vi "TLB Native Dynamic Events ver 0.26.vi"() -> ()   [LabVIEW 2018] (continued)
              shift-right: [w366] -> w361
              shift-left: w362 -> [w365]
              tunnel: string[] ["STOP", "RESET ENCODERS", "RESET YAW", "RESET ARM", "RESET ALL SENSORS", "DISPOSE CAM BUFFERS", "DISPOSE PROC BUFFERS", "CAM CLOSE", ""] -> [w364] mode=indexing
              n203 = Enqueue Element(queue=w365, element=w364) -> (queue out=w366:refnum<queue>)  [unwired: 2 in, 2 out]
            }
          }
          frame 4, Default {
            # ">>> Motor control cluster >>>"
            # ">>> yStepper command>>>"
            n204 = Dequeue Element(queue=w378, timeout in ms (-1)=w377, error in (no error)=w373) -> (element=w376:T8)  [unwired: 3 out]
            n205 = case shown="\"Start Task 5\"" w376 {
              tunnel: [w381 w389 w397 w405 w413 w421 w429 w437 w445 w452 w462 w470 w477 w480] -> w372
              tunnel: w375 -> [w382 w390 w398 w406 w414 w422 w430 w438 w446 w453 w461 w469 w477 w481]
              tunnel: [State_Type_Definitions,_for_0.26g_versions_and_later_2."Task 1A" ("Enum") State_Type_Definitions,_for_0.26g_versions_and_later_2."Task 2:Raise Arm" ("Enum") State_Type_Definitions,_for_0.26g_versions_and_later_2."Task 3" ("Enum") State_Type_Definitions,_for_0.26g_versions_and_later_2."Task 4_A" ("Enum") State_Type_Definitions,_for_0.26g_versions_and_later_2."Task 5A" ("Enum") State_Type_Definitions,_for_0.26g_versions_and_later_2."Task 6_A" ("Enum") State_Type_Definitions,_for_0.26g_versions_and_later_2."Task 8A: RAISE ARM" ("Enum") State_Type_Definitions,_for_0.26g_versions_and_later_2."Task 8A: RAISE ARM" ("Enum") State_Type_Definitions,_for_0.26g_versions_and_later_2."Task 8A: RAISE ARM" ("Enum") State_Type_Definitions,_for_0.26g_versions_and_later_2."Task 8A: RAISE ARM" ("Enum") State_Type_Definitions,_for_0.26g_versions_and_later_2."Task 9A: Raise Arm" ("Enum") State_Type_Definitions."Task 9F: SCAN IMAGE" ("Enum") State_Type_Definitions,_for_0.26g_versions_and_later_2."Idle" ("Enum") State_Type_Definitions,_for_0.26g_versions_and_later_2."Shutdown" ("Enum")] -> w374
              tunnel: [enum16{"Ball", "Soap", "Gel", "Pipe", "None"}."None" ("Object recognition mode") enum16{"Ball", "Soap", "Gel", "Pipe", "None"}."None" ("Object recognition mode") enum16{"Ball", "Soap", "Gel", "Pipe", "None"}."None" ("Object recognition mode") enum16{"Ball", "Soap", "Gel", "Pipe", "None"}."None" ("Object recognition mode") enum16{"Ball", "Soap", "Gel", "Pipe", "None"}."None" ("Object recognition mode") enum16{"Ball", "Soap", "Gel", "Pipe", "None"}."None" ("Object recognition mode") enum16{"Ball", "Soap", "Gel", "Pipe", "None"}."Ball" ("Object recognition mode") enum16{"Ball", "Soap", "Gel", "Pipe", "None"}."Gel" ("Object recognition mode") enum16{"Ball", "Soap", "Gel", "Pipe", "None"}."Pipe" ("Object recognition mode") enum16{"Ball", "Soap", "Gel", "Pipe", "None"}."Soap" ("Object recognition mode") enum16{"Ball", "Soap", "Gel", "Pipe", "None"}."None" ("Object recognition mode") enum16{"Ball", "Soap", "Gel", "Pipe", "None"}."None" ("Object recognition mode") enum16{"Ball", "Soap", "Gel", "Pipe", "None"}."None" ("Object recognition mode") enum16{"Ball", "Soap", "Gel", "Pipe", "None"}."None" ("Object recognition mode")] -> w367
              frame "Start Task 1" {
                n206 = for {
                  shift-right: [w386] -> w381
                  shift-left: w382 -> [w385]
                  tunnel: string[] ["RESET ENCODERS", "RESET YAW", "FORWARD", "READ ENCODERS"] -> [w384] mode=indexing
                  n207 = Enqueue Element(queue=w385, element=w384) -> (queue out=w386:refnum<queue>)  [unwired: 2 in, 2 out]
                }
              }
              frame "Start Task 2" {
                n208 = for {
                  shift-right: [w394] -> w389
                  shift-left: w390 -> [w393]
                  tunnel: string[] ["RESET ENCODERS", "RESET YAW", "READ ULTRASONIC", "ARDUINO - ULTRASONIC"] -> [w392] mode=indexing
                  n209 = Enqueue Element(queue=w393, element=w392) -> (queue out=w394:refnum<queue>)  [unwired: 2 in, 2 out]
                }
              }
              frame "Start Task 3" {
                n210 = for {
                  shift-right: [w402] -> w397
                  shift-left: w398 -> [w401]
                  tunnel: string[] ["RESET ENCODERS", "READ ENCODERS", "R-ACW"] -> [w400] mode=indexing
                  n211 = Enqueue Element(queue=w401, element=w400) -> (queue out=w402:refnum<queue>)  [unwired: 2 in, 2 out]
                }
              }
              frame "Start Task 4" {
                n212 = for {
                  shift-right: [w410] -> w405
                  shift-left: w406 -> [w409]
                  tunnel: string[] ["RESET YAW", "RESET ENCODERS", "RESET ARM", "RESET FLAGS", "", ""] -> [w408] mode=indexing
                  n213 = Enqueue Element(queue=w409, element=w408) -> (queue out=w410:refnum<queue>)  [unwired: 2 in, 2 out]
                }
              }
              frame "Start Task 5" {
                n214 = for {
                  shift-right: [w418] -> w413
                  shift-left: w414 -> [w417]
                  tunnel: string[] ["RESET YAW", "RESET ENCODERS", "RESET ARM", "RESET ALL SENSORS", "", ""] -> [w416] mode=indexing
                  n215 = Enqueue Element(queue=w417, element=w416) -> (queue out=w418:refnum<queue>)  [unwired: 2 in, 2 out]
                }
              }
              frame "Start Task 6" {
                n216 = for {
                  shift-right: [w426] -> w421
                  shift-left: w422 -> [w425]
                  tunnel: string[] ["OPEN LOG CAM ", "", "", "", "", ""] -> [w424] mode=indexing
                  n217 = Enqueue Element(queue=w425, element=w424) -> (queue out=w426:refnum<queue>)  [unwired: 2 in, 2 out]
                }
              }
              frame "Start Task 8 - BALL" {
                n218 = for {
                  shift-right: [w434] -> w429
                  shift-left: w430 -> [w433]
                  tunnel: string[] ["RESET YAW", "RESET ENCODERS", "RESET ARM", "RESET FLAGS"] -> [w432] mode=indexing
                  n219 = Enqueue Element(queue=w433, element=w432) -> (queue out=w434:refnum<queue>)  [unwired: 2 in, 2 out]
                }
              }
              frame "Start Task 8 - Gel" {
                n220 = for {
                  shift-right: [w442] -> w437
                  shift-left: w438 -> [w441]
                  tunnel: string[] ["RESET YAW", "RESET ENCODERS", "RESET ARM", "RESET FLAGS"] -> [w440] mode=indexing
                  n221 = Enqueue Element(queue=w441, element=w440) -> (queue out=w442:refnum<queue>)  [unwired: 2 in, 2 out]
                }
              }
              frame "Start Task 8 - Pipe" {
                n222 = for {
                  shift-right: [w450] -> w445
                  shift-left: w446 -> [w449]
                  tunnel: string[] ["RESET YAW", "RESET ENCODERS", "RESET ARM", "RESET FLAGS"] -> [w448] mode=indexing
                  n223 = Enqueue Element(queue=w449, element=w448) -> (queue out=w450:refnum<queue>)  [unwired: 2 in, 2 out]
                }
              }
              frame "Start Task 8 - Soap" {
                n224 = for {
                  shift-right: [w458] -> w452
                  shift-left: w453 -> [w457]
                  tunnel: string[] ["RESET YAW", "RESET ENCODERS", "RESET ARM", "RESET FLAGS"] -> [w456] mode=indexing
                  n225 = Enqueue Element(queue=w457, element=w456) -> (queue out=w458:refnum<queue>)  [unwired: 2 in, 2 out]
                }
              }
              frame "Start Task 9" {
                n226 = for {
                  shift-right: [w466] -> w462
                  shift-left: w461 -> [w465]
                  tunnel: string[] ["RESET ENCODERS", "READ ENCODERS", "Z STEPPER BOX HEIGHT"] -> [w464] mode=indexing
                  n227 = Enqueue Element(queue=w465, element=w464) -> (queue out=w466:refnum<queue>)  [unwired: 2 in, 2 out]
                }
              }
              frame "Start Task A" {
                n228 = for {
                  shift-right: [w474] -> w470
                  shift-left: w469 -> [w473]
                  tunnel: string[] ["RESET ENCODERS", "READ ENCODERS", "RESET YAW", "Z STEPPER BOX HEIGHT"] -> [w472] mode=indexing
                  n229 = Enqueue Element(queue=w473, element=w472) -> (queue out=w474:refnum<queue>)  [unwired: 2 in, 2 out]
                }
              }
              frame "None", Default {
              }
              frame "Exit" {
                n230 = for {
                  shift-right: [w485] -> w480
                  shift-left: w481 -> [w484]
                  tunnel: string[] ["STOP", "RESET ENCODERS", "RESET YAW", "EXIT"] -> [w483] mode=indexing
                  n231 = Enqueue Element(queue=w484, element=w483) -> (queue out=w485:refnum<queue>)  [unwired: 2 in, 2 out]
                }
              }
            }
          }
          frame 5 {
            # ">> Item Selection Bias >>"
            # ">>> yStepper command>>>"
            n232 = for {
              shift-right: [w496] -> w490
              shift-left: w492 -> [w495]
              tunnel: string[] ["INIT", "RESET ENCODERS", "RESET FLAGS", "CAM CLOSE", "DISPOSE BUFFERS", "EXIT", ""] -> [w494] mode=indexing
              n233 = Enqueue Element(queue=w495, element=w494) -> (queue out=w496:refnum<queue>)  [unwired: 2 in, 2 out]
            }
          }
          frame 6 {
            # ">>> Motor control cluster >>>"
            # ">> Line detection >>"
            # ">> Checks if 1 metre moved >>"
            # ">>> yStepper command>>>"
            # "Use 250"
            n234 = Greater?(x=w506, y=265.0) -> (0:w500:bool)
            n235 = Dequeue Element(queue=w513, timeout in ms (-1)=w512, error in (no error)=w511) -> (element=w510:T8)  [unwired: 3 out]
            n236 = And(x=w499, y=w500) -> (x .and. y?=w497:bool)
            n237 = case shown="\"Start Task 1\", Default" w510 {
              tunnel: w498 -> [w514 _]
              tunnel: [w524 State_Type_Definitions,_for_0.26g_versions_and_later_2."True Stop" ("Enum")] -> w509
              tunnel: w508 -> [w522 w539]
              tunnel: [w521 w538] -> w507
              tunnel: [State_Type_Definitions,_for_0.26g_versions_and_later_2."Idle" ("Enum") State_Type_Definitions,_for_0.26g_versions_and_later_2."Shutdown" ("Enum")] -> w504
              tunnel: w497 -> [w515 _]
              frame "Start Task 1", Default {
                n238 = Or(x=w515, y=w514) -> (x .or. y?=w516:bool)
                n239 = case shown="True" w516 {
                  tunnel: w522 -> [w527 w533]
                  tunnel: [w526 w531] -> w521
                  frame False {
                    n240 = for {
                      shift-right: [w529] -> w526
                      shift-left: w527 -> [w530]
                      tunnel: string[] ["READ ENCODERS", "READ NAVX", "FORWARD", "READ LINE SENSOR"] ("element") -> [w528] mode=indexing
                      n241 = Enqueue Element(queue=w530, element=w528) -> (queue out=w529:refnum<queue>)  [unwired: 2 in, 2 out]
                    }
                  }
                  frame True {
                    n242 = for {
                      shift-right: [w535] -> w531
                      shift-left: w533 -> [w536]
                      tunnel: string[] ["RESET YAW", "RESET ENCODERS", "STOP", ""] -> [w534] mode=indexing
                      n243 = Enqueue Element(queue=w536, element=w534) -> (queue out=w535:refnum<queue>)  [unwired: 2 in, 2 out]
                    }
                  }
                }
                n244 = Select(t=State_Type_Definitions,_for_0.26g_versions_and_later_2."True Stop" ("Enum"), s=w514, f=State_Type_Definitions,_for_0.26g_versions_and_later_2."Task 1B" ("Enum")) -> (s? t:f=w519:T16)
                n245 = Select(t=w519, s=w515, f=State_Type_Definitions,_for_0.26g_versions_and_later_2."Task 1A" ("Enum")) -> (s? t:f=w524:T16)
              }
              frame "Exit" {
                n246 = for {
                  shift-right: [w543] -> w538
                  shift-left: w539 -> [w544]
                  tunnel: string[] ["STOP", "RESET ENCODERS", "RESET YAW", ""] -> [w542] mode=indexing
                  n247 = Enqueue Element(queue=w544, element=w542) -> (queue out=w543:refnum<queue>)  [unwired: 2 in, 2 out]
                }
              }
            }
          }
          frame 7 {
            # ">>> Motor control cluster >>>"
            # ">> Line detection >>"
            # ">> Adds small distance overhead after 1M >>"
            # ">>> yStepper command>>>"
            n248 = Greater?(x=w551, y=50.0) -> (0:w545:bool)
            n249 = Dequeue Element(queue=w560, timeout in ms (-1)=w559, error in (no error)=w558) -> (element=w557:T8)  [unwired: 3 out]
            n250 = Or(x=w545, y=w552) -> (x .or. y?=w556:bool)
            n251 = case shown="\"Start Task 1\", Default" w557 {
              tunnel: w556 -> [w563 _]
              tunnel: [w567 State_Type_Definitions,_for_0.26g_versions_and_later_2."True Stop" ("Enum")] -> w555
              tunnel: w554 -> [w564 w582]
              tunnel: [w562 w581] -> w553
              tunnel: [State_Type_Definitions,_for_0.26g_versions_and_later_2."Idle" ("Enum") State_Type_Definitions,_for_0.26g_versions_and_later_2."Shutdown" ("Enum")] -> w549
              frame "Start Task 1", Default {
                n252 = case shown="True" w563 {
                  tunnel: w564 -> [w570 w576]
                  tunnel: [w569 w574] -> w562
                  frame False {
                    n253 = for {
                      shift-right: [w572] -> w569
                      shift-left: w570 -> [w573]
                      tunnel: string[] ["READ ENCODERS", "READ NAVX", "FORWARD", "READ LINE SENSOR"] ("element") -> [w571] mode=indexing
                      n254 = Enqueue Element(queue=w573, element=w571) -> (queue out=w572:refnum<queue>)  [unwired: 2 in, 2 out]
                    }
                  }
                  frame True {
                    n255 = for {
                      shift-right: [w578] -> w574
                      shift-left: w576 -> [w579]
                      tunnel: string[] ["RESET YAW", "RESET ENCODERS", "STOP", ""] -> [w577] mode=indexing
                      n256 = Enqueue Element(queue=w579, element=w577) -> (queue out=w578:refnum<queue>)  [unwired: 2 in, 2 out]
                    }
                  }
                }
                n257 = Select(t=State_Type_Definitions,_for_0.26g_versions_and_later_2."True Stop" ("Enum"), s=w563, f=State_Type_Definitions,_for_0.26g_versions_and_later_2."Task 1B" ("Enum")) -> (s? t:f=w567:T16)
              }
              frame "Exit" {
                n258 = for {
                  shift-right: [w586] -> w581
                  shift-left: w582 -> [w587]
                  tunnel: string[] ["STOP", "RESET ENCODERS", "RESET YAW", ""] -> [w585] mode=indexing
                  n259 = Enqueue Element(queue=w587, element=w585) -> (queue out=w586:refnum<queue>)  [unwired: 2 in, 2 out]
                }
              }
            }
          }
          frame 8 {
            # ">> Stepper height reeached >>"
            # ">>> yStepper command>>>"
            # ">> Manual override >>"
            n260 = Dequeue Element(queue=w593, timeout in ms (-1)=w592, error in (no error)=w591) -> (element=w602:T8)  [unwired: 3 out]
            n261 = Equal?(x=w595, y=u8 60) -> (x = y?=w600:bool)
            n262 = case shown="\"Start Task 1\", Default" w602 {
              tunnel: [w613 State_Type_Definitions,_for_0.26g_versions_and_later_2."True Stop" ("Enum")] -> w597
              tunnel: [w611 w628] -> w590
              tunnel: w599 -> [w610 _]
              tunnel: w598 -> [w604 _]
              tunnel: [State_Type_Definitions,_for_0.26g_versions_and_later_2."Idle" ("Enum") State_Type_Definitions,_for_0.26g_versions_and_later_2."Shutdown" ("Enum")] -> w596
              tunnel: w600 -> [w603 _]
              frame "Start Task 1", Default {
                # ">> WIill proceed to part ii if not manual override >>"
                # ">>If ENABLE or Trigger is set to true>>"
                n263 = Or(x=w603, y=w604) -> (x .or. y?=w605:bool)
                n264 = case shown="True" w603 {
                  tunnel: [w616 w622] -> w611
                  tunnel: w610 -> [w615 w621]
                  frame False {
                    n265 = for {
                      shift-right: [w618] -> w616
                      shift-left: w615 -> [w619]
                      tunnel: string[] ["Z STEPPER CAM HEIGHT", "READ STEPPER VALUES"] ("element") -> [w617] mode=indexing
                      n266 = Enqueue Element(queue=w619, element=w617) -> (queue out=w618:refnum<queue>)  [unwired: 2 in, 2 out]
                    }
                  }
                  frame True {
                    n267 = for {
                      shift-right: [w624] -> w622
                      shift-left: w621 -> [w625]
                      tunnel: string[] ["ARDUINO - ULTRASONIC", "READ ULTRASONIC", "", "", "", ""] -> [w623] mode=indexing
                      n268 = Enqueue Element(queue=w625, element=w623) -> (queue out=w624:refnum<queue>)  [unwired: 2 in, 2 out]
                    }
                  }
                }
                n269 = Select(t=State_Type_Definitions,_for_0.26g_versions_and_later_2."True Stop" ("Enum"), s=w604, f=State_Type_Definitions,_for_0.26g_versions_and_later_2."Task 2:Sensor Mode" ("Enum")) -> (s? t:f=w607:T16)
                n270 = Select(t=w607, s=w605, f=State_Type_Definitions,_for_0.26g_versions_and_later_2."Task 2:Raise Arm" ("Enum")) -> (s? t:f=w613:T16)
              }
              frame "Exit" {
                n271 = for {
                  shift-right: [w631] -> w628
                  shift-left: _ -> [w632]
                  tunnel: string[] ["STOP", "RESET ENCODERS", "RESET YAW", ""] -> [w630] mode=indexing
                  n272 = Enqueue Element(queue=w632, element=w630) -> (queue out=w631:refnum<queue>)  [unwired: 2 in, 2 out]
                }
              }
            }
          }
          frame 9 {
            w649 = u8 20 ("y")
            # ">>> yStepper command>>>"
            # ">>Object detected>>"
            n273 = Dequeue Element(queue=w642, timeout in ms (-1)=w641, error in (no error)=w640) -> (element=w650:T8)  [unwired: 3 out]
            n274 = Less?(x=w638, y=w649) -> (x < y?=w648:bool)
            n275 = Less?(x=w637, y=w649) -> (x < y?=w647:bool)
            n276 = Or(x=w648, y=w647) -> (x .or. y?=w633:bool)
            n277 = case shown="\"Start Task 1\", Default" w650 {
              tunnel: w633 -> [w653 _]
              tunnel: [w660 State_Type_Definitions,_for_0.26g_versions_and_later_2."True Stop" ("Enum")] -> w646
              tunnel: w639 -> [w652 _]
              tunnel: w643 -> [w659 w676]
              tunnel: [w658 w677] -> w645
              tunnel: [State_Type_Definitions,_for_0.26g_versions_and_later_2."Idle" ("Enum") State_Type_Definitions,_for_0.26g_versions_and_later_2."Shutdown" ("Enum")] -> w644
              frame "Start Task 1", Default {
                n278 = case shown="False" w653 {
                  tunnel: w659 -> [w663 w670]
                  tunnel: [w664 w669] -> w658
                  frame False {
                    n279 = for {
                      tunnel: string[] ["READ ULTRASONIC", "STOP"] ("element") -> [w665] mode=indexing
                      shift-right: [w667] -> w664
                      shift-left: w663 -> [w666]
                      n280 = Enqueue Element(queue=w666, element=w665) -> (queue out=w667:refnum<queue>)  [unwired: 2 in, 2 out]
                    }
                  }
                  frame True {
                    n281 = for {
                      shift-right: [w672] -> w669
                      shift-left: w670 -> [w673]
                      tunnel: string[] ["RESET ENCODERS", "READ NAVX", "READ ENCODERS"] -> [w671] mode=indexing
                      n282 = Enqueue Element(queue=w673, element=w671) -> (queue out=w672:refnum<queue>)  [unwired: 2 in, 2 out]
                    }
                  }
                }
                n283 = Or(x=w653, y=w652) -> (x .or. y?=w651:bool)
                n284 = Select(t=State_Type_Definitions,_for_0.26g_versions_and_later_2."True Stop" ("Enum"), s=w652, f=State_Type_Definitions,_for_0.26g_versions_and_later_2."Task 2:Reverse Mode" ("Enum")) -> (s? t:f=w654:T16)
                n285 = Select(t=w654, s=w651, f=State_Type_Definitions,_for_0.26g_versions_and_later_2."Task 2:Sensor Mode" ("Enum")) -> (s? t:f=w660:T16)
              }
              frame "Exit" {
                n286 = for {
                  shift-right: [w680] -> w677
                  shift-left: w676 -> [w681]
                  tunnel: string[] ["STOP", "RESET ENCODERS", "RESET YAW", "ARDUINO MODE 0"] -> [w679] mode=indexing
                  n287 = Enqueue Element(queue=w681, element=w679) -> (queue out=w680:refnum<queue>)  [unwired: 2 in, 2 out]
                }
              }
            }
          }
          frame 10 {
            # ">>> yStepper command>>>"
            n288 = Dequeue Element(queue=w692, timeout in ms (-1)=w693, error in (no error)=w694) -> (element=w696:T8)  [unwired: 3 out]
            n289 = Less?(x=w686, y=-50.0) -> (x < y?=w684:bool)
            n290 = case shown="\"Start Task 1\", Default" w696 {
              tunnel: [w706 State_Type_Definitions,_for_0.26g_versions_and_later_2."True Stop" ("Enum")] -> w688
              tunnel: w695 -> [w699 _]
              tunnel: w691 -> [w705 w722]
              tunnel: [w704 w723] -> w687
              tunnel: [State_Type_Definitions,_for_0.26g_versions_and_later_2."Idle" ("Enum") State_Type_Definitions,_for_0.26g_versions_and_later_2."Shutdown" ("Enum")] -> w689
              tunnel: w684 -> [w697 _]
              frame "Start Task 1", Default {
                n291 = case shown="True" w697 {
                  tunnel: w705 -> [w709 w716]
                  tunnel: [w710 w715] -> w704
                  frame False {
                    n292 = for {
                      tunnel: string[] ["READ ENCODERS", "REVERSE", "READ NAVX"] ("element") -> [w711] mode=indexing
                      shift-right: [w713] -> w710
                      shift-left: w709 -> [w712]
                      n293 = Enqueue Element(queue=w712, element=w711) -> (queue out=w713:refnum<queue>)  [unwired: 2 in, 2 out]
                    }
                  }
                  frame True {
                    n294 = for {
                      shift-right: [w718] -> w715
                      shift-left: w716 -> [w719]
                      tunnel: string[] ["STOP", "ARDUINO - ULTRASONIC", "READ ULTRASONIC", "RESET ENCODERS"] -> [w717] mode=indexing
                      n295 = Enqueue Element(queue=w719, element=w717) -> (queue out=w718:refnum<queue>)  [unwired: 2 in, 2 out]
                    }
                  }
                }
                n296 = Or(x=w697, y=w699) -> (x .or. y?=w698:bool)
                n297 = Select(t=State_Type_Definitions,_for_0.26g_versions_and_later_2."True Stop" ("Enum"), s=w699, f=State_Type_Definitions,_for_0.26g_versions_and_later_2."Task 2:Sensor Mode" ("Enum")) -> (s? t:f=w700:T16)
                n298 = Select(t=w700, s=w698, f=State_Type_Definitions,_for_0.26g_versions_and_later_2."Task 2:Reverse Mode" ("Enum")) -> (s? t:f=w706:T16)
              }
              frame "Exit" {
                n299 = for {
                  shift-right: [w726] -> w723
                  shift-left: w722 -> [w727]
                  tunnel: string[] ["STOP", "RESET ENCODERS", "RESET YAW", "ARDUINO MODE 0"] -> [w725] mode=indexing
                  n300 = Enqueue Element(queue=w727, element=w725) -> (queue out=w726:refnum<queue>)  [unwired: 2 in, 2 out]
                }
              }
            }
          }
          frame 11 {
            # ">>> Motor control cluster >>>"
            # ">>> yStepper command>>>"
            n301 = Dequeue Element(queue=w743, timeout in ms (-1)=w742, error in (no error)=w741) -> (element=w732:T8)  [unwired: 3 out]
            n302 = Less?(x=w740, y=-160.0) -> (x < y?=w737:bool)
            n303 = Or(x=w737, y=w738) -> (x .or. y?=w733:bool)
            n304 = case shown="\"Start Task 1\", Default" w732 {
              tunnel: w733 -> [w746 _]
              tunnel: [w750 State_Type_Definitions,_for_0.26g_versions_and_later_2."True Stop" ("Enum")] -> w734
              tunnel: w736 -> [w747 w766]
              tunnel: [w745 w765] -> w735
              tunnel: [State_Type_Definitions,_for_0.26g_versions_and_later_2."Idle" ("Enum") State_Type_Definitions,_for_0.26g_versions_and_later_2."Shutdown" ("Enum")] -> w731
              frame "Start Task 1", Default {
                n305 = case shown="False" w746 {
                  tunnel: w747 -> [w753 w759]
                  tunnel: [w752 w757] -> w745
                  frame False {
                    n306 = for {
                      shift-right: [w755] -> w752
                      shift-left: w753 -> [w756]
                      tunnel: string[] ["READ ENCODERS", "R-CW"] ("element") -> [w754] mode=indexing
                      n307 = Enqueue Element(queue=w756, element=w754) -> (queue out=w755:refnum<queue>)  [unwired: 2 in, 2 out]
                    }
                  }
                  frame True {
                    n308 = for {
                      shift-right: [w761] -> w757
                      shift-left: w759 -> [w762]
                      tunnel: string[] ["RESET YAW", "RESET ENCODERS", "STOP", "ARDUINO MODE 0"] -> [w760] mode=indexing
                      n309 = Enqueue Element(queue=w762, element=w760) -> (queue out=w761:refnum<queue>)  [unwired: 2 in, 2 out]
                    }
                  }
                }
                n310 = Select(t=State_Type_Definitions,_for_0.26g_versions_and_later_2."True Stop" ("Enum"), s=w746, f=State_Type_Definitions,_for_0.26g_versions_and_later_2."Task 3" ("Enum")) -> (s? t:f=w750:T16)
              }
              frame "Exit" {
                n311 = for {
                  shift-right: [w769] -> w765
                  shift-left: w766 -> [w770]
                  tunnel: string[] ["STOP", "RESET ENCODERS", "RESET YAW", ""] -> [w768] mode=indexing
                  n312 = Enqueue Element(queue=w770, element=w768) -> (queue out=w769:refnum<queue>)  [unwired: 2 in, 2 out]
                }
              }
            }
          }
          frame 12 {
            # ">> Stepper height reeached >>"
            # ">>> yStepper command>>>"
            # ">> Manual override >>"
            n313 = Dequeue Element(queue=w784, timeout in ms (-1)=w783, error in (no error)=w782) -> (element=w781:T8)  [unwired: 3 out]
            n314 = Equal?(x=w775, y=u8 60) -> (x = y?=w773:bool)
            n315 = case shown="\"Start Task 1\", Default" w781 {
              tunnel: [w796 State_Type_Definitions,_for_0.26g_versions_and_later_2."True Stop" ("Enum")] -> w780
              tunnel: [w794 w812] -> w779
              tunnel: w785 -> [w793 w809]
              tunnel: w778 -> [w787 _]
              tunnel: [State_Type_Definitions,_for_0.26g_versions_and_later_2."Idle" ("Enum") State_Type_Definitions,_for_0.26g_versions_and_later_2."Shutdown" ("Enum")] -> w777
              tunnel: w773 -> [w786 _]
              frame "Start Task 1", Default {
                # ">> WIill proceed to part ii if not manual override >>"
                # ">>If ENABLE or Trigger is set to true>>"
                n316 = Or(x=w786, y=w787) -> (x .or. y?=w788:bool)
                n317 = case shown="False" w786 {
                  tunnel: [w799 w805] -> w794
                  tunnel: w793 -> [w798 w804]
                  frame False {
                    n318 = for {
                      shift-right: [w801] -> w799
                      shift-left: w798 -> [w802]
                      tunnel: string[] ["Z STEPPER CAM HEIGHT", "READ STEPPER VALUES"] ("element") -> [w800] mode=indexing
                      n319 = Enqueue Element(queue=w802, element=w800) -> (queue out=w801:refnum<queue>)  [unwired: 2 in, 2 out]
                    }
                  }
                  frame True {
                    n320 = for {
                      shift-right: [w807] -> w805
                      shift-left: w804 -> [w808]
                      tunnel: string[] ["ARDUINO - ULTRASONIC", "READ ULTRASONIC", "FORWARD", "", "", ""] -> [w806] mode=indexing
                      n321 = Enqueue Element(queue=w808, element=w806) -> (queue out=w807:refnum<queue>)  [unwired: 2 in, 2 out]
                    }
                  }
                }
                n322 = Select(t=State_Type_Definitions,_for_0.26g_versions_and_later_2."True Stop" ("Enum"), s=w787, f=State_Type_Definitions,_for_0.26g_versions_and_later_2."Task 4_B" ("Enum")) -> (s? t:f=w790:T16)
                n323 = Select(t=w790, s=w788, f=State_Type_Definitions,_for_0.26g_versions_and_later_2."Task 4_A" ("Enum")) -> (s? t:f=w796:T16)
              }
              frame "Exit" {
                n324 = for {
                  shift-right: [w815] -> w812
                  shift-left: w809 -> [w816]
                  tunnel: string[] ["STOP", "RESET ENCODERS", "RESET YAW", ""] -> [w814] mode=indexing
                  n325 = Enqueue Element(queue=w816, element=w814) -> (queue out=w815:refnum<queue>)  [unwired: 2 in, 2 out]
                }
              }
            }
          }
          frame 13 {
            w822 = u8 20
            # ">> Path blocked >>"
            # ">>> yStepper command>>>"
            # ">> Manual override >>"
            n326 = Dequeue Element(queue=w831, timeout in ms (-1)=w830, error in (no error)=w829) -> (element=w828:T8)  [unwired: 3 out]
            n327 = Less?(x=w824, y=w822) -> (x < y?=w819:bool)
            n328 = Less?(x=w823, y=w822) -> (x < y?=w820:bool)
            n329 = And(x=w820, y=w819) -> (x .and. y?=w821:bool)
            n330 = case shown="\"Start Task 1\", Default" w828 {
              tunnel: [w845 State_Type_Definitions,_for_0.26g_versions_and_later_2."True Stop" ("Enum")] -> w833
              tunnel: [w843 w860] -> w834
              tunnel: w827 -> [w842 _]
              tunnel: w832 -> [w836 _]
              tunnel: [State_Type_Definitions,_for_0.26g_versions_and_later_2."Idle" ("Enum") State_Type_Definitions,_for_0.26g_versions_and_later_2."Shutdown" ("Enum")] -> w826
              tunnel: w821 -> [w835 _]
              frame "Start Task 1", Default {
                # ">> Manual override forces program to true stop >>"
                # ">>If ENABLE or Trigger is set to true>>"
                n331 = Or(x=w835, y=w836) -> (x .or. y?=w841:bool)
                n332 = case shown="False" w835 {
                  tunnel: [w848 w853] -> w843
                  tunnel: w842 -> [w847 w852]
                  frame False {
                    n333 = for {
                      shift-right: [w850] -> w848
                      shift-left: w847 -> [w851]
                      tunnel: string[] ["FORWARD", "READ ULTRASONIC", "READ NAVX"] ("element") -> [w849] mode=indexing
                      n334 = Enqueue Element(queue=w851, element=w849) -> (queue out=w850:refnum<queue>)  [unwired: 2 in, 2 out]
                    }
                  }
                  frame True {
                    n335 = for {
                      shift-right: [w856] -> w853
                      shift-left: w852 -> [w857]
                      tunnel: string[] ["STOP", "RESET YAW", "RESET ENCODERS", "RESET FLAGS"] -> [w855] mode=indexing
                      n336 = Enqueue Element(queue=w857, element=w855) -> (queue out=w856:refnum<queue>)  [unwired: 2 in, 2 out]
                    }
                  }
                }
                n337 = Select(t=State_Type_Definitions,_for_0.26g_versions_and_later_2."True Stop" ("Enum"), s=w836, f=State_Type_Definitions,_for_0.26g_versions_and_later_2."Task 4_C" ("Enum")) -> (s? t:f=w838:T16)
                n338 = Select(t=w838, s=w841, f=State_Type_Definitions,_for_0.26g_versions_and_later_2."Task 4_B" ("Enum")) -> (s? t:f=w845:T16)
              }
              frame "Exit" {
                n339 = for {
                  shift-right: [w863] -> w860
                  shift-left: _ -> [w864]
                  tunnel: string[] ["STOP", "RESET ENCODERS", "RESET YAW", ""] -> [w862] mode=indexing
                  n340 = Enqueue Element(queue=w864, element=w862) -> (queue out=w863:refnum<queue>)  [unwired: 2 in, 2 out]
                }
              }
            }
          }
          frame 14 {
            w876 = u8 20
            # ">> xDistance travelled>>"
            # ">> Path NOT blocked >>"
            # ">>> yStepper command>>>"
            # ">> Manual override >>"
            n341 = Dequeue Element(queue=w886, timeout in ms (-1)=w879, error in (no error)=w878) -> (element=w880:T8)  [unwired: 3 out]
            n342 = Greater?(x=w868, y=w876) -> (0:w874:bool)
            n343 = Greater?(x=w873, y=80.0) -> (0:w871:bool)
            n344 = Greater?(x=w867, y=w876) -> (0:w875:bool)
            n345 = And(x=w875, y=w874) -> (x .and. y?=w870:bool)
            n346 = And(x=w871, y=w870) -> (x .and. y?=w869:bool)
            n347 = case shown="\"Start Task 1\", Default" w880 {
              tunnel: [w897 State_Type_Definitions,_for_0.26g_versions_and_later_2."True Stop" ("Enum")] -> w883
              tunnel: [w895 w913] -> w882
              tunnel: w885 -> [w894 w910]
              tunnel: w884 -> [w888 _]
              tunnel: [State_Type_Definitions,_for_0.26g_versions_and_later_2."Idle" ("t") State_Type_Definitions,_for_0.26g_versions_and_later_2."Shutdown" ("Enum")] -> w881
              tunnel: w869 -> [w887 _]
              frame "Start Task 1", Default {
                # ">> Manual override forces program to true stop >>"
                # ">>If ENABLE or Trigger is set to true>>"
                n348 = Or(x=w887, y=w888) -> (x .or. y?=w893:bool)
                n349 = case shown="False" w887 {
                  tunnel: [w900 w905] -> w895
                  tunnel: w894 -> [w898 w904]
                  frame False {
                    n350 = for {
                      shift-right: [w902] -> w900
                      shift-left: w898 -> [w903]
                      tunnel: string[] ["RIGHT", "READ NAVX", "READ ENCODERS", "READ ULTRASONIC"] ("element") -> [w901] mode=indexing
                      n351 = Enqueue Element(queue=w903, element=w901) -> (queue out=w902:refnum<queue>)  [unwired: 2 in, 2 out]
                    }
                  }
                  frame True {
                    n352 = for {
                      shift-right: [w908] -> w905
                      shift-left: w904 -> [w909]
                      tunnel: string[] ["STOP", "RESET YAW", "RESET ENCODERS", "ARDUINO - ULTRASONIC"] -> [w907] mode=indexing
                      n353 = Enqueue Element(queue=w909, element=w907) -> (queue out=w908:refnum<queue>)  [unwired: 2 in, 2 out]
                    }
                  }
                }
                n354 = Select(t=State_Type_Definitions,_for_0.26g_versions_and_later_2."True Stop" ("Enum"), s=w888, f=State_Type_Definitions,_for_0.26g_versions_and_later_2."Task 4_D" ("Enum")) -> (s? t:f=w889:T16)
                n355 = Select(t=w889, s=w893, f=State_Type_Definitions,_for_0.26g_versions_and_later_2."Task 4_C" ("Enum")) -> (s? t:f=w897:T16)
              }
              frame "Exit" {
                n356 = for {
                  shift-right: [w916] -> w913
                  shift-left: w910 -> [w917]
                  tunnel: string[] ["STOP", "RESET ENCODERS", "RESET YAW", ""] -> [w915] mode=indexing
                  n357 = Enqueue Element(queue=w917, element=w915) -> (queue out=w916:refnum<queue>)  [unwired: 2 in, 2 out]
                }
              }
            }
          }
          frame 15 {
            w940 = u8 20
            # ">>> Motor control cluster >>>"
            # ">> Line detected >>"
            # ">> yDistance travelled>>"
            # ">> Path blocked >>"
            # ">>> yStepper command>>>"
            # ">> Manual override >>"
            n358 = Less?(x=w925, y=w940) -> (x < y?=w938:bool)
            n359 = Greater?(x=w929, y=200.0) -> (0:w936:bool)
            n360 = Less?(x=w924, y=w940) -> (x < y?=w939:bool)
            n361 = And(x=w939, y=w938) -> (x .and. y?=w935:bool)
            n362 = Dequeue Element(queue=w932, timeout in ms (-1)=w931, error in (no error)=w930) -> (element=w941:T8)  [unwired: 3 out]
            n363 = Or(x=w936, y=w935) -> (x .or. y?=w919:bool)
            n364 = And(x=w920, y=w919) -> (x .and. y?=w918:bool)
            n365 = case shown="\"Start Task 1\", Default" w941 {
              tunnel: [w952 State_Type_Definitions,_for_0.26g_versions_and_later_2."True Stop" ("Enum")] -> w928
              tunnel: [w950 w968] -> w926
              tunnel: w933 -> [w949 w965]
              tunnel: w934 -> [w943 _]
              tunnel: [State_Type_Definitions,_for_0.26g_versions_and_later_2."Idle" ("t") State_Type_Definitions,_for_0.26g_versions_and_later_2."Shutdown" ("Enum")] -> w927
              tunnel: w918 -> [w942 _]
              frame "Start Task 1", Default {
                # ">> Manual override forces program to true stop >>"
                # ">>If ENABLE or Trigger is set to true>>"
                n366 = Or(x=w942, y=w943) -> (x .or. y?=w948:bool)
                n367 = case shown="False" w942 {
                  tunnel: [w955 w960] -> w950
                  tunnel: w949 -> [w953 w959]
                  frame False {
                    n368 = for {
                      shift-right: [w957] -> w955
                      shift-left: w953 -> [w958]
                      tunnel: string[] ["FORWARD", "READ NAVX", "READ ENCODERS", "READ ULTRASONIC", "READ LINE SENSOR"] ("element") -> [w956] mode=indexing
                      n369 = Enqueue Element(queue=w958, element=w956) -> (queue out=w957:refnum<queue>)  [unwired: 2 in, 2 out]
                    }
                  }
                  frame True {
                    n370 = for {
                      shift-right: [w963] -> w960
                      shift-left: w959 -> [w964]
                      tunnel: string[] ["STOP", "RESET YAW", "RESET ENCODERS", "RESET FLAGS"] -> [w962] mode=indexing
                      n371 = Enqueue Element(queue=w964, element=w962) -> (queue out=w963:refnum<queue>)  [unwired: 2 in, 2 out]
                    }
                  }
                }
                n372 = Select(t=State_Type_Definitions,_for_0.26g_versions_and_later_2."True Stop" ("Enum"), s=w943, f=State_Type_Definitions,_for_0.26g_versions_and_later_2."True Stop" ("Enum")) -> (s? t:f=w944:T16)
                n373 = Select(t=w944, s=w948, f=State_Type_Definitions,_for_0.26g_versions_and_later_2."Task 4_D" ("Enum")) -> (s? t:f=w952:T16)
              }
              frame "Exit" {
                n374 = for {
                  shift-right: [w971] -> w968
                  shift-left: w965 -> [w972]
                  tunnel: string[] ["STOP", "RESET ENCODERS", "RESET YAW", ""] -> [w970] mode=indexing
                  n375 = Enqueue Element(queue=w972, element=w970) -> (queue out=w971:refnum<queue>)  [unwired: 2 in, 2 out]
                }
              }
            }
          }
          frame 16 {
            # "Stays in Task 5_A until stepper reaches desired \nheight"
            # ">>> Motor control cluster >>>"
            # ">>> yStepper command>>>"
            # ">> Manual override >>"
            n376 = Dequeue Element(queue=w983, timeout in ms (-1)=w982, error in (no error)=w984) -> (element=w981:T8)  [unwired: 3 out]
            n377 = Equal?(x=w980, y=u8 1) -> (x = y?=w978:bool)
            n378 = case shown="\"Start Task 1\", Default" w981 {
              tunnel: [w994 State_Type_Definitions,_for_0.26g_versions_and_later_2."True Stop" ("Enum")] -> w985
              tunnel: [w997 w1014] -> w986
              tunnel: [State_Type_Definitions,_for_0.26g_versions_and_later_2."Idle" ("Enum") State_Type_Definitions,_for_0.26g_versions_and_later_2."Shutdown" ("Enum")] -> w987
              tunnel: w978 -> [w993 _]
              tunnel: w977 -> [w992 _]
              tunnel: w976 -> [w988 w1011]
              frame "Start Task 1", Default {
                # "T: Go back to idle, F: Continue with task\""
                # ">> Manual override >>"
                n379 = case shown="True" w993 {
                  tunnel: [w1001 w1007] -> w997
                  tunnel: w988 -> [w999 w1005]
                  frame False {
                    n380 = for {
                      tunnel: string[] ["Z STEPPER GRAB HEIGHT", "READ STEPPER VALUES"] ("element") -> [w1002] mode=indexing
                      shift-right: [w1004] -> w1001
                      shift-left: w999 -> [w1003]
                      n381 = Enqueue Element(queue=w1003, element=w1002) -> (queue out=w1004:refnum<queue>)  [unwired: 2 in, 2 out]
                    }
                  }
                  frame True {
                    n382 = for {
                      shift-right: [w1009] -> w1007
                      shift-left: w1005 -> [w1010]
                      tunnel: string[] ["SET TIMER 2", "", ""] -> [w1008] mode=indexing
                      n383 = Enqueue Element(queue=w1010, element=w1008) -> (queue out=w1009:refnum<queue>)  [unwired: 2 in, 2 out]
                    }
                  }
                }
                n384 = Or(x=w993, y=w992) -> (x .or. y?=w995:bool)
                n385 = Select(t=State_Type_Definitions,_for_0.26g_versions_and_later_2."True Stop" ("Enum"), s=w992, f=State_Type_Definitions,_for_0.26g_versions_and_later_2."Task 5B" ("Enum")) -> (s? t:f=w989:T16)
                n386 = Select(t=w989, s=w995, f=State_Type_Definitions,_for_0.26g_versions_and_later_2."Task 5A" ("Enum")) -> (s? t:f=w994:T16)
              }
              frame "Exit" {
                n387 = for {
                  shift-right: [w1017] -> w1014
                  shift-left: w1011 -> [w1018]
                  tunnel: string[] ["STOP", "RESET ENCODERS", "RESET YAW", "ARDUINO MODE 0"] -> [w1016] mode=indexing
                  n388 = Enqueue Element(queue=w1018, element=w1016) -> (queue out=w1017:refnum<queue>)  [unwired: 2 in, 2 out]
                }
              }
            }
          }
          frame 17 {
            # ">>> yStepper command>>>"
            n389 = Dequeue Element(queue=w1025, timeout in ms (-1)=w1024, error in (no error)=w1026) -> (element=w1023:T8)  [unwired: 3 out]
            n390 = case shown="\"Start Task 1\", Default" w1023 {
              tunnel: [w1038 State_Type_Definitions,_for_0.26g_versions_and_later_2."True Stop" ("Enum")] -> w1028
              tunnel: [w1041 w1058] -> w1027
              tunnel: [State_Type_Definitions,_for_0.26g_versions_and_later_2."Idle" ("Enum") State_Type_Definitions,_for_0.26g_versions_and_later_2."Shutdown" ("Enum")] -> w1029
              tunnel: w1031 -> [w1037 _]
              tunnel: w1030 -> [w1033 w1055]
              tunnel: w1019 -> [w1032 _]
              frame "Start Task 1", Default {
                # "T: Go back to idle, F: Continue with task\""
                # ">> Manual override >>"
                n391 = case shown="True" w1032 {
                  tunnel: [w1045 w1051] -> w1041
                  tunnel: w1033 -> [w1043 w1049]
                  frame False {
                    n392 = for {
                      tunnel: string[] ["CLOSE CLAW", "START TIMER", ""] ("element") -> [w1046] mode=indexing
                      shift-right: [w1048] -> w1045
                      shift-left: w1043 -> [w1047]
                      n393 = Enqueue Element(queue=w1047, element=w1046) -> (queue out=w1048:refnum<queue>)  [unwired: 2 in, 2 out]
                    }
                  }
                  frame True {
                    n394 = for {
                      shift-right: [w1053] -> w1051
                      shift-left: w1049 -> [w1054]
                      tunnel: string[] ["STOP", "", "", ""] -> [w1052] mode=indexing
                      n395 = Enqueue Element(queue=w1054, element=w1052) -> (queue out=w1053:refnum<queue>)  [unwired: 2 in, 2 out]
                    }
                  }
                }
                n396 = Or(x=w1032, y=w1037) -> (x .or. y?=w1039:bool)
                n397 = Select(t=State_Type_Definitions,_for_0.26g_versions_and_later_2."True Stop" ("Enum"), s=w1037, f=State_Type_Definitions,_for_0.26g_versions_and_later_2."Task 5C" ("Enum")) -> (s? t:f=w1034:T16)
                n398 = Select(t=w1034, s=w1039, f=State_Type_Definitions,_for_0.26g_versions_and_later_2."Task 5B" ("Enum")) -> (s? t:f=w1038:T16)
              }
              frame "Exit" {
                n399 = for {
                  shift-right: [w1061] -> w1058
                  shift-left: w1055 -> [w1062]
                  tunnel: string[] ["STOP", "RESET ENCODERS", "RESET YAW", "ARDUINO MODE 0"] -> [w1060] mode=indexing
                  n400 = Enqueue Element(queue=w1062, element=w1060) -> (queue out=w1061:refnum<queue>)  [unwired: 2 in, 2 out]
                }
              }
            }
          }
          frame 18 {
            # ">>> Motor control cluster >>>"
            # ">>> yStepper command>>>"
            # ">> Manual override >>"
            n401 = Equal?(x=w1065, y=u8 60) -> (x = y?=w1063:bool)
            n402 = Dequeue Element(queue=w1075, timeout in ms (-1)=w1074, error in (no error)=w1073) -> (element=w1072:T8)  [unwired: 3 out]
            n403 = case shown="\"Start Task 1\", Default" w1072 {
              tunnel: [w1084 State_Type_Definitions,_for_0.26g_versions_and_later_2."True Stop" ("Enum")] -> w1077
              tunnel: [w1087 w1104] -> w1070
              tunnel: [State_Type_Definitions,_for_0.26g_versions_and_later_2."Idle" ("Enum") State_Type_Definitions,_for_0.26g_versions_and_later_2."Shutdown" ("Enum")] -> w1069
              tunnel: w1071 -> [w1078 _]
              tunnel: w1076 -> [w1083 w1101]
              tunnel: w1063 -> [w1082 _]
              frame "Start Task 1", Default {
                # ">> Is time up? >>"
                # "Determines if object is in range to pick up"
                # ">> Manual override >>"
                n404 = case shown="True" w1082 {
                  tunnel: [w1091 w1097] -> w1087
                  tunnel: w1083 -> [w1089 w1095]
                  frame False {
                    n405 = for {
                      tunnel: string[] ["Z STEPPER CAM HEIGHT", "READ STEPPER VALUES"] ("element") -> [w1092] mode=indexing
                      shift-right: [w1094] -> w1091
                      shift-left: w1089 -> [w1093]
                      n406 = Enqueue Element(queue=w1093, element=w1092) -> (queue out=w1094:refnum<queue>)  [unwired: 2 in, 2 out]
                    }
                  }
                  frame True {
                    n407 = for {
                      shift-right: [w1099] -> w1097
                      shift-left: w1095 -> [w1100]
                      tunnel: string[] ["SET TIMER 5", "", ""] -> [w1098] mode=indexing
                      n408 = Enqueue Element(queue=w1100, element=w1098) -> (queue out=w1099:refnum<queue>)  [unwired: 2 in, 2 out]
                    }
                  }
                }
                n409 = Or(x=w1082, y=w1078) -> (x .or. y?=w1085:bool)
                n410 = Select(t=State_Type_Definitions,_for_0.26g_versions_and_later_2."True Stop" ("Enum"), s=w1078, f=State_Type_Definitions,_for_0.26g_versions_and_later_2."Task 5D" ("Enum")) -> (s? t:f=w1080:T16)